vi "Dresden R2R Sputter 03.02.2018 IY24.vi"() -> ()   [LabVIEW 2009] (continued)
                                n16803 = local write "Semi"(TRUE ("Semi")) -> ()
                                }
                                }
                                n16804 = local read "Ch1_Ch_atm_di"() -> (w27011:bool)
                                n16805 = case shown="False" w27011 {
                                tunnel: [w27018 TRUE] -> w27013
                                frame #0 {
                                n16806 = local read "Ch1_Ch_vbv_di"() -> (w27019:bool)
                                n16807 = case shown="False" w27019 {
                                tunnel: [FALSE TRUE] -> w27018
                                frame #0 {
                                n16808 = Wait Until Next ms Multiple(millisecond multiple=u32 200) -> ()  [unwired: 1 out]
                                n16809 = local write "Ch1_Ch_vbv_do"(TRUE ("Ch1_Ch_cc_on_off_di")) -> ()
                                }
                                frame #1 {
                                }
                                }
                                }
                                frame #1 {
                                }
                                }
                                n16810 = local read "Semi"() -> (w27014:bool)
                                n16811 = Or(x=w27013, y=w27014) -> (x .or. y?=w27012:bool)
                                }
                                }
                                frame #1 {
                                }
                                }
                                }
                                frame #2 {
                                n16812 = local read "Semi"() -> (w27027:bool)
                                n16813 = case shown="False" w27027 {
                                frame #0 {
                                n16814 = local write "Ch1_Sd10"(TRUE ("Ch1_Sd9")) -> ()
                                n16815 = Wait (ms)(milliseconds to wait=u32 1000) -> ()  [unwired: 1 out]
                                }
                                frame #1 {
                                }
                                }
                                }
                                }
                                }
                                frame #1 {
                                }
                                }
                                }
                                }
                              }
                              frame #11 {
                                # "CH-VBV CLOSE &  CHECK"
                                n16816 = local read "Yes"() -> (w27030:bool)
                                n16817 = case shown="True" w27030 {
                                frame #0 {
                                }
                                frame #1 {
                                n16818 = local read "Semi"() -> (w27031:bool)
                                n16819 = case shown="False" w27031 {
                                frame #0 {
                                n16820 = stacked-sequence {
                                frame #0 {
                                n16821 = local read "Semi"() -> (w27032:bool)
                                n16822 = case shown="False" w27032 {
                                frame #0 {
                                n16823 = while {
                                i -> [w27040]
                                stop <- w27036 stop-if-true
                                n16824 = Greater?(x=w27040, y=50) -> (0:w27039:bool)
                                n16825 = case shown="True" w27039 {
                                frame #0 {
                                }
                                frame #1 {
                                n16826 = local write "Error Message"("Shut Down Process  cancelled\nbecause  CH-VBV  not closed.\nPlease check CH-VBV1 connections." ("Error Message")) -> ()
                                n16827 = local write "Semi"(TRUE ("Semi")) -> ()
                                }
                                }
                                n16828 = local read "Tp1_speed_gui"() -> (w27034:i32)
                                n16829 = Greater Or Equal?(x=w27034, y=u64 100) -> (x >= y?=w27033:bool)
                                n16830 = case shown="True" w27033 {
                                tunnel: [TRUE w27043] -> w27037
                                frame #0 {
                                }
                                frame #1 {
                                n16831 = local read "Ch1_Ch_vbv_di"() -> (w27044:bool)
                                n16832 = case shown="True" w27044 {
                                tunnel: [TRUE FALSE] -> w27043
                                frame #0 {
                                }
                                frame #1 {
                                n16833 = Wait Until Next ms Multiple(millisecond multiple=u32 500) -> ()  [unwired: 1 out]
                                n16834 = local write "Ch1_Ch_vbv_do"(FALSE ("Ch1_Ch_cc_on_off_di")) -> ()
                                }
                                }
                                }
                                }
                                n16835 = local read "Semi"() -> (w27038:bool)
                                n16836 = Or(x=w27037, y=w27038) -> (x .or. y?=w27036:bool)
                                }
                                }
                                frame #1 {
                                }
                                }
                                }
                                frame #1 {
                                n16837 = local read "Semi"() -> (w27051:bool)
                                n16838 = case shown="False" w27051 {
                                frame #0 {
                                n16839 = local write "Ch1_Sd11"(TRUE ("Ch1_Sd13")) -> ()
                                n16840 = Wait (ms)(milliseconds to wait=u32 1000) -> ()  [unwired: 1 out]
                                }
                                frame #1 {
                                }
                                }
                                }
                                frame #2 {
                                n16841 = local read "Semi"() -> (w27054:bool)
                                n16842 = case shown="False" w27054 {
                                frame #0 {
                                n16843 = Wait (ms)(milliseconds to wait=u32 3000) -> ()  [unwired: 1 out]
                                }
                                frame #1 {
                                }
                                }
                                }
                                }
                                }
                                frame #1 {
                                }
                                }
                                }
                                }
                              }
                              frame #12 {
                                # "CH-VBV OPEN &  CHECK"
                                n16844 = local read "Yes"() -> (w27056:bool)
                                n16845 = case shown="True" w27056 {
                                frame #0 {
                                }
                                frame #1 {
                                n16846 = local read "Semi"() -> (w27057:bool)
                                n16847 = case shown="False" w27057 {
                                frame #0 {
                                n16848 = stacked-sequence {
                                frame #0 {
                                n16849 = local read "Semi"() -> (w27058:bool)
                                n16850 = case shown="False" w27058 {
                                frame #0 {
                                n16851 = while {
                                i -> [w27064]
                                stop <- w27060 stop-if-true
                                n16852 = Greater?(x=w27064, y=200) -> (0:w27063:bool)
                                n16853 = case shown="True" w27063 {
                                frame #0 {
                                }
                                frame #1 {
                                n16854 = local write "Error Message"("Shut Down Process  cancelled\nbecause  CH-VBV  not opened.\nPlease check CH-VBV1 connections." ("Error Message")) -> ()
                                n16855 = local write "Semi"(TRUE ("Semi")) -> ()
                                }
                                }
                                n16856 = local read "Ch1_Ch_vbv_di"() -> (w27059:bool)
                                n16857 = case shown="False" w27059 {
                                tunnel: [FALSE TRUE] -> w27061
                                frame #0 {
                                n16858 = local write "Ch1_Ch_vbv_do"(TRUE ("Ch1_Ch_cc_on_off_di")) -> ()
                                n16859 = Wait Until Next ms Multiple(millisecond multiple=u32 500) -> ()  [unwired: 1 out]
                                }
                                frame #1 {
                                }
                                }
                                n16860 = local read "Semi"() -> (w27062:bool)
                                n16861 = Or(x=w27061, y=w27062) -> (x .or. y?=w27060:bool)
                                }
                                }
                                frame #1 {
                                }
                                }
                                }
                                frame #1 {
                                n16862 = local read "Semi"() -> (w27072:bool)
                                n16863 = case shown="False" w27072 {
                                frame #0 {
                                n16864 = local write "Ch1_Sd12"(TRUE ("Ch1_Sd12")) -> ()
                                n16865 = Wait (ms)(milliseconds to wait=u32 1000) -> ()  [unwired: 1 out]
                                }
                                frame #1 {
                                }
                                }
                                }
                                }
                                }
                                frame #1 {
                                }
                                }
                                }
                                }
                              }
                              frame #13 {
                                # "TRNS GV-BP2 OPEN"
                                n16866 = local read "Yes"() -> (w27075:bool)
                                n16867 = case shown="True" w27075 {
                                frame #0 {
                                }
                                frame #1 {
                                n16868 = local read "Semi"() -> (w27076:bool)
                                n16869 = case shown="False" w27076 {
                                frame #0 {
                                n16870 = stacked-sequence {
                                frame #0 {
                                n16871 = local read "Semi"() -> (w27077:bool)
                                n16872 = case shown="False" w27077 {
                                frame #0 {
                                n16873 = while {
                                i -> [w27085]
                                stop <- w27082 stop-if-true
                                n16874 = Greater?(x=w27085, y=800) -> (0:w27084:bool)
                                n16875 = case shown="True" w27084 {
                                frame #0 {
                                }
                                frame #1 {
                                n16876 = local write "Error Message"("Shut Down process was cancelled.\nPlease check Trns GV-BP2\n connections." ("Error Message")) -> ()
                                n16877 = local write "Semi"(TRUE ("Semi")) -> ()
                                }
                                }
                                n16878 = local read "Ch1_pressure"() -> (w27080:dbl)
                                n16879 = Greater Or Equal?(x=w27080, y=700.0) -> (x >= y?=w27078:bool)
                                n16880 = case shown="False" w27078 {
                                tunnel: [FALSE w27089] -> w27081
                                frame #0 {
                                n16881 = Wait Until Next ms Multiple(millisecond multiple=u32 500) -> ()  [unwired: 1 out]
                                }
                                frame #1 {
                                n16882 = local read "Ch1_Trns_gv_bp2_di"() -> (w27090:bool)
                                n16883 = case shown="False" w27090 {
                                tunnel: [FALSE TRUE] -> w27089
                                frame #0 {
                                n16884 = local write "Ch1_Trns_gv_bp2_do"(TRUE ("Ch1_Trns_gv_bp2_do")) -> ()
                                n16885 = Wait Until Next ms Multiple(millisecond multiple=u32 500) -> ()  [unwired: 1 out]
                                }
                                frame #1 {
                                }
                                }
                                }
                                }
                                n16886 = local read "Semi"() -> (w27083:bool)
                                n16887 = Or(x=w27081, y=w27083) -> (x .or. y?=w27082:bool)
                                }
                                }
                                frame #1 {
                                }
                                }
                                }
                                frame #1 {
                                n16888 = local read "Semi"() -> (w27097:bool)
                                n16889 = case shown="False" w27097 {
                                frame #0 {
                                n16890 = Wait (ms)(milliseconds to wait=u32 1000) -> ()  [unwired: 1 out]
                                n16891 = local write "Ch1_Sd13"(TRUE ("Ch1_Sd12")) -> ()
                                }
                                frame #1 {
                                }
                                }
                                }
                                frame #2 {
                                n16892 = local read "Semi"() -> (w27100:bool)
                                n16893 = case shown="False" w27100 {
                                frame #0 {
                                n16894 = Wait (ms)(milliseconds to wait=u32 2000) -> ()  [unwired: 1 out]
                                }
                                frame #1 {
                                }
                                }
                                }
                                }
                                }
                                frame #1 {
                                }
                                }
                                }
                                }
                              }
                              frame #14 {
                                # "CH-ATM OPEN &  CHECK"
                                n16895 = local read "Yes"() -> (w27102:bool)
                                n16896 = case shown="True" w27102 {
                                frame #0 {
                                }
                                frame #1 {
                                n16897 = local read "Semi"() -> (w27103:bool)
                                n16898 = case shown="False" w27103 {
                                frame #0 {
                                n16899 = stacked-sequence {
                                frame #0 {
                                n16900 = local read "Semi"() -> (w27104:bool)
                                n16901 = case shown="False" w27104 {
                                frame #0 {
                                n16902 = while {
                                i -> [w27110]
                                stop <- w27107 stop-if-true
                                n16903 = Greater?(x=w27110, y=1700) -> (0:w27109:bool)
                                n16904 = case shown="True" w27109 {
                                frame #0 {
                                }
                                frame #1 {
                                n16905 = local write "Error Message"("Shut Down process was cancelled.\nPlease check Chamber \nvacuum connections." ("Error Message")) -> ()
                                n16906 = local write "Semi"(TRUE ("Semi")) -> ()
                                }
                                }
                                n16907 = local read "Ch1_Ch_atm_di"() -> (w27106:bool)
                                n16908 = case shown="False" w27106 {
                                tunnel: [FALSE TRUE] -> w27105
                                frame #0 {
                                n16909 = Wait Until Next ms Multiple(millisecond multiple=u32 500) -> ()  [unwired: 1 out]
                                }
                                frame #1 {
                                }
                                }
                                n16910 = local read "Semi"() -> (w27108:bool)
                                n16911 = Or(x=w27105, y=w27108) -> (x .or. y?=w27107:bool)
                                }
                                }
                                frame #1 {
                                }
                                }
                                }
                                frame #1 {
                                n16912 = local read "Semi"() -> (w27117:bool)
                                n16913 = case shown="False" w27117 {
                                frame #0 {
                                n16914 = local write "Ch1_Sd14"(TRUE ("Ch1_Sd10")) -> ()
                                n16915 = Wait (ms)(milliseconds to wait=u32 1000) -> ()  [unwired: 1 out]
                                }
                                frame #1 {
                                }
                                }
                                }
                                frame #2 {
                                n16916 = local read "Semi"() -> (w27120:bool)
                                n16917 = case shown="False" w27120 {
                                frame #0 {
                                n16918 = Wait (ms)(milliseconds to wait=u32 2000) -> ()  [unwired: 1 out]
                                }
                                frame #1 {
                                }
                                }
                                }
                                }
                                }
                                frame #1 {
                                }
                                }
                                }
                                }
                              }
                              frame #15 {
                                # "TRNS GV-BP2 OPEN"
                                n16919 = local read "Semi"() -> (w27122:bool)
                                n16920 = case shown="False" w27122 {
                                frame #0 {
                                n16921 = stacked-sequence {
                                frame #0 {
                                n16922 = local read "Semi"() -> (w27123:bool)
                                n16923 = case shown="False" w27123 {
                                frame #0 {
                                n16924 = while {
                                i -> [w27129]
                                stop <- w27125 stop-if-true
                                n16925 = Greater?(x=w27129, y=50) -> (0:w27128:bool)
                                n16926 = case shown="True" w27128 {
                                frame #0 {
                                }
                                frame #1 {
                                n16927 = local write "Error Message"("Shut Down Process  cancelled\nbecause  Trns-GV-BP2  not closed.\nPlease check Trns-GV-BP2  connections." ("Error Message")) -> ()
                                n16928 = local write "Semi"(TRUE ("Semi")) -> ()
                                }
                                }
                                n16929 = local read "Ch1_Trns_gv_bp2_di"() -> (w27124:bool)
                                n16930 = case shown="True" w27124 {
                                tunnel: [TRUE FALSE] -> w27126
                                frame #0 {
                                }
                                frame #1 {
                                n16931 = Wait Until Next ms Multiple(millisecond multiple=u32 500) -> ()  [unwired: 1 out]
                                n16932 = local write "Ch1_Trns_gv_bp2_do"(FALSE ("Ch1_Ch_cc_on_off_di")) -> ()
                                }
                                }
                                n16933 = local read "Semi"() -> (w27127:bool)
                                n16934 = Or(x=w27126, y=w27127) -> (x .or. y?=w27125:bool)
                                }
                                }
                                frame #1 {
                                }
                                }
                                }
                                frame #1 {
                                n16935 = local read "Semi"() -> (w27137:bool)
                                n16936 = case shown="False" w27137 {
                                frame #0 {
                                n16937 = local write "Ch1_Sd15"(TRUE ("Ch1_Sd10 3")) -> ()
                                n16938 = Wait (ms)(milliseconds to wait=u32 1000) -> ()  [unwired: 1 out]
                                }
                                frame #1 {
                                }
                                }
                                }
                                }
                                }
                                frame #1 {
                                }
                                }
                              }
                              frame #16 {
                                # "CH-VBV CLOSE &  CHECK"
                                n16939 = local read "Yes"() -> (w27140:bool)
                                n16940 = case shown="True" w27140 {
                                frame #0 {
                                }
                                frame #1 {
                                n16941 = local read "Semi"() -> (w27141:bool)
                                n16942 = case shown="False" w27141 {
                                frame #0 {
                                n16943 = stacked-sequence {
                                frame #0 {
                                n16944 = local read "Semi"() -> (w27142:bool)
                                n16945 = case shown="False" w27142 {
                                frame #0 {
                                n16946 = while {
                                i -> [w27152]
                                stop <- w27148 stop-if-true
                                n16947 = Greater?(x=w27152, y=50) -> (0:w27151:bool)
                                n16948 = case shown="True" w27151 {
                                frame #0 {
                                }
                                frame #1 {
                                n16949 = local write "Error Message"("Shut Down Process  cancelled\nbecause  CH-VBV  not closed.\nPlease check CH-VBV1 connections." ("Error Message")) -> ()
                                n16950 = local write "Semi"(TRUE ("Semi")) -> ()
                                }
                                }
                                n16951 = local read "Tp1_speed_gui"() -> (w27146:i32)
                                n16952 = local read "Yes"() -> (w27145:bool)
                                n16953 = Greater Or Equal?(x=w27146, y=u64 100) -> (x >= y?=w27144:bool)
                                n16954 = And(x=w27145, y=w27144) -> (x .and. y?=w27143:bool)
                                n16955 = case shown="True" w27143 {
                                tunnel: [TRUE w27155] -> w27149
                                frame #0 {
                                }
                                frame #1 {
                                n16956 = local read "Ch1_Ch_vbv_di"() -> (w27156:bool)
                                n16957 = case shown="False" w27156 {
                                tunnel: [TRUE FALSE] -> w27155
                                frame #0 {
                                }
                                frame #1 {
                                n16958 = Wait Until Next ms Multiple(millisecond multiple=u32 500) -> ()  [unwired: 1 out]
                                n16959 = local write "Ch1_Ch_vbv_do"(FALSE ("Ch1_Ch_cc_on_off_di")) -> ()
                                }
                                }
                                }
                                }
                                n16960 = local read "Semi"() -> (w27150:bool)
                                n16961 = Or(x=w27149, y=w27150) -> (x .or. y?=w27148:bool)
                                }
                                }
                                frame #1 {
                                }
                                }
                                }
                                frame #1 {
                                n16962 = local read "Semi"() -> (w27163:bool)
                                n16963 = case shown="False" w27163 {
                                frame #0 {
                                n16964 = local write "Ch1_Sd16"(TRUE ("Ch1_Sd10 2")) -> ()
                                n16965 = Wait (ms)(milliseconds to wait=u32 1000) -> ()  [unwired: 1 out]
                                }
                                frame #1 {
                                }
                                }
                                }
                                frame #2 {
                                n16966 = local read "Semi"() -> (w27166:bool)
                                n16967 = case shown="False" w27166 {
                                frame #0 {
                                n16968 = Wait (ms)(milliseconds to wait=u32 3000) -> ()  [unwired: 1 out]
                                }
                                frame #1 {
                                }
                                }
                                }
                                }
                                }
                                frame #1 {
                                }
                                }
                                }
                                }
                              }
                              frame #17 {
                                # "CLOSE PC-BV"
                                n16969 = local read "Yes"() -> (w27168:bool)
                                n16970 = case shown="True" w27168 {
                                frame #0 {
                                }
                                frame #1 {
                                n16971 = local read "Semi"() -> (w27169:bool)
                                n16972 = case shown="False" w27169 {
                                frame #0 {
                                n16973 = stacked-sequence {
                                frame #0 {
                                n16974 = local read "Semi"() -> (w27170:bool)
                                n16975 = case shown="False" w27170 {
                                frame #0 {
                                n16976 = stacked-sequence {
                                frame #0 {
                                n16977 = local read "Semi"() -> (w27171:bool)
                                n16978 = case shown="False" w27171 {
                                frame #0 {
                                n16979 = local write "Pc_bv1_auto_close"(TRUE ("Tp1_auto_start")) -> ()
                                }
                                frame #1 {
                                }
                                }
                                }
                                frame #1 {
                                n16980 = local read "Semi"() -> (w27173:bool)
                                n16981 = case shown="False" w27173 {
                                frame #0 {
                                n16982 = Wait (ms)(milliseconds to wait=u32 1000) -> ()  [unwired: 1 out]
                                }
                                frame #1 {
                                }
                                }
                                }
                                frame #2 {
                                n16983 = local read "Semi"() -> (w27175:bool)
                                n16984 = case shown="False" w27175 {
                                frame #0 {
                                n16985 = while {
                                i -> [w27181]
                                stop <- w27177 stop-if-true
                                n16986 = local read "Pc_bv_closed_ch1"() -> (w27179:bool)
                                n16987 = Greater?(x=w27181, y=120) -> (0:w27180:bool)
                                n16988 = local read "Semi"() -> (w27178:bool)
                                n16989 = Compound Arithmetic op=OR(w27178, w27179, w27180) -> (w27177:bool)
                                n16990 = Wait (ms)(milliseconds to wait=u32 500) -> ()  [unwired: 1 out]
                                }
                                }
                                frame #1 {
                                }
                                }
                                }
                                frame #3 {
                                n16991 = local read "Semi"() -> (w27183:bool)
                                n16992 = case shown="False" w27183 {
                                frame #0 {
                                n16993 = local read "Pc_bv_closed_ch1"() -> (w27184:bool)
                                n16994 = case shown="False" w27184 {
                                frame #0 {
                                n16995 = local write "Pc_bv1_auto_close"(TRUE ("Pc_bv1_auto_open")) -> ()
                                }
                                frame #1 {
                                }
                                }
                                }
                                frame #1 {
                                }
                                }
                                }
                                frame #4 {
                                n16996 = local read "Semi"() -> (w27186:bool)
                                n16997 = case shown="False" w27186 {
                                frame #0 {
                                n16998 = local read "Pc_bv_closed_ch1"() -> (w27187:bool)
                                n16999 = case shown="False" w27187 {
                                frame #0 {
                                n17000 = Wait (ms)(milliseconds to wait=u32 1000) -> ()  [unwired: 1 out]
                                }
                                frame #1 {
                                }
                                }
                                }
                                frame #1 {
                                }
                                }
                                }
                                frame #5 {
                                n17001 = local read "Semi"() -> (w27189:bool)
                                n17002 = case shown="False" w27189 {
                                frame #0 {
                                n17003 = while {
                                i -> [w27195]
                                stop <- w27191 stop-if-true
                                n17004 = local read "Pc_bv_closed_ch1"() -> (w27193:bool)
                                n17005 = Greater?(x=w27195, y=120) -> (0:w27194:bool)
                                n17006 = local read "Semi"() -> (w27192:bool)
                                n17007 = Compound Arithmetic op=OR(w27192, w27193, w27194) -> (w27191:bool)
                                n17008 = Wait (ms)(milliseconds to wait=u32 500) -> ()  [unwired: 1 out]
                                }
                                }
                                frame #1 {
                                }
                                }
                                }
                                frame #6 {
                                n17009 = local read "Semi"() -> (w27197:bool)
                                n17010 = case shown="False" w27197 {
                                frame #0 {
                                n17011 = local read "Pc_bv_closed_ch1"() -> (w27198:bool)
                                n17012 = case shown="False" w27198 {
                                frame #0 {
                                n17013 = local write "Error Message"("Shut Down process  cancelled\nbecause  PC-BV not closed.\nPlease check PC-BV1 connections." ("Error Message")) -> ()
                                n17014 = Wait (ms)(milliseconds to wait=u32 1000) -> ()  [unwired: 1 out]
                                }
                                frame #1 {
                                }
                                }
                                }
                                frame #1 {
                                }
                                }
                                }
                                }
                                }
                                frame #1 {
                                }
                                }
                                }
                                frame #1 {
                                n17015 = local read "Semi"() -> (w27201:bool)
                                n17016 = case shown="False" w27201 {
                                frame #0 {
                                n17017 = Wait (ms)(milliseconds to wait=u32 1000) -> ()  [unwired: 1 out]
                                n17018 = local write "Ch1_Sd17"(TRUE ("Ch1_Sd14")) -> ()
                                }
                                frame #1 {
                                }
                                }
                                }
                                }
                                }
                                frame #1 {
                                }
                                }
                                }
                                }
                              }
                              frame #18 {
                                # "CH-VBV CLOSE &  CHECK"
                                n17019 = local read "Semi"() -> (w27204:bool)
                                n17020 = case shown="False" w27204 {
                                frame #0 {
                                n17021 = stacked-sequence {
                                frame #0 {
                                n17022 = local read "Semi"() -> (w27205:bool)
                                n17023 = case shown="False" w27205 {
                                frame #0 {
                                n17024 = while {
                                i -> [w27211]
                                stop <- w27207 stop-if-true
                                n17025 = Greater?(x=w27211, y=50) -> (0:w27210:bool)
                                n17026 = case shown="True" w27210 {
                                frame #0 {
                                }
                                frame #1 {
                                n17027 = local write "Error Message"("Shut Down Process  cancelled\nbecause  CH-VBV  not closed.\nPlease check CH-VBV1 connections." ("Error Message")) -> ()
                                n17028 = local write "Semi"(TRUE ("Semi")) -> ()
                                }
                                }
                                n17029 = local read "Ch1_Ch_vbv_di"() -> (w27206:bool)
                                n17030 = case shown="True" w27206 {
                                tunnel: [TRUE FALSE] -> w27208
                                frame #0 {
                                }
                                frame #1 {
                                n17031 = Wait Until Next ms Multiple(millisecond multiple=u32 500) -> ()  [unwired: 1 out]
                                n17032 = local write "Ch1_Ch_vbv_do"(FALSE ("Ch1_Ch_cc_on_off_di")) -> ()
                                }
                                }
                                n17033 = local read "Semi"() -> (w27209:bool)
                                n17034 = Or(x=w27208, y=w27209) -> (x .or. y?=w27207:bool)
                                }
                                }
                                frame #1 {
                                }
                                }
                                }
                                frame #1 {
                                n17035 = local read "Semi"() -> (w27219:bool)
                                n17036 = case shown="False" w27219 {
                                frame #0 {
                                n17037 = local write "Ch1_Sd18"(TRUE ("Ch1_Sd10 3")) -> ()
                                n17038 = Wait (ms)(milliseconds to wait=u32 1000) -> ()  [unwired: 1 out]
                                }
                                frame #1 {
                                }
                                }
                                }
                                }
                                }
                                frame #1 {
                                }
                                }
                              }
                              frame #19 {
                                # "FINISH SHUTDOWN"
                                n17039 = local read "Semi"() -> (w27222:bool)
                                n17040 = case shown="False" w27222 {
                                frame #0 {
                                n17041 = stacked-sequence {
                                frame #0 {
                                n17042 = local read "Semi"() -> (w27223:bool)
                                n17043 = case shown="False" w27223 {
                                frame #0 {
                                w27224 = TRUE ("Visible")
                                n17044 = property on="final_mes_tab" class="TabCtl (strict)"("Visible"=w27224) -> ()  [unwired: 2 in, 2 out]
                                n17045 = local write "Cnt_Do_Buzzer"(w27224) -> ()
                                n17046 = local write "system_status"("Shut Down Process was completed." ("system_status")) -> ()
                                n17047 = Wait (ms)(milliseconds to wait=u32 3000) -> ()  [unwired: 1 out]
                                }
                                frame #1 {
                                }
                                }
                                }
                                frame #1 {
                                n17048 = local read "Semi"() -> (w27227:bool)
                                n17049 = case shown="False" w27227 {
                                frame #0 {
                                w27230 = FALSE ("Visible")
                                n17050 = property on="final_mes_tab" class="TabCtl (strict)"("Visible"=w27230) -> ()  [unwired: 2 in, 2 out]
                                n17051 = local write "Shutdown_ch1"(w27230) -> ()
                                n17052 = local write "Cnt_Do_Buzzer"(w27230) -> ()
                                n17053 = local write "system_status"("" ("system_status")) -> ()
                                n17054 = Wait (ms)(milliseconds to wait=u32 3000) -> ()  [unwired: 1 out]
                                }
                                frame #1 {
                                }
                                }
                                }
                                frame #2 {
                                n17055 = local read "Semi"() -> (w27231:bool)
                                n17056 = case shown="False" w27231 {
                                frame #0 {
                                n17057 = stacked-sequence {
                                frame #0 {
                                n17058 = local write "Pps_code_entry"("PF233=" ("Pps_code_entry")) -> ()
                                }
                                frame #1 {
                                n17059 = Wait (ms)(milliseconds to wait=u32 500) -> ()  [unwired: 1 out]
                                }
                                frame #2 {
                                n17060 = local write "Ppsok"(TRUE ("Ppsok")) -> ()
                                }
                                frame #3 {
                                n17061 = Wait (ms)(milliseconds to wait=u32 500) -> ()  [unwired: 1 out]
                                }
                                }
                                }
                                frame #1 {
                                }
                                }
                                }
                                frame #3 {
                                n17062 = local read "Semi"() -> (w27236:bool)
                                n17063 = case shown="False" w27236 {
                                frame #0 {
                                n17064 = stacked-sequence {
                                frame #0 {
                                n17065 = local write "Pps_code_entry"("PF234=" ("Pps_code_entry")) -> ()
                                }
                                frame #1 {
                                n17066 = Wait (ms)(milliseconds to wait=u32 500) -> ()  [unwired: 1 out]
                                }
                                frame #2 {
                                n17067 = local write "Ppsok"(TRUE ("Ppsok")) -> ()
                                }
                                frame #3 {
                                n17068 = Wait (ms)(milliseconds to wait=u32 500) -> ()  [unwired: 1 out]
                                }
                                }
                                }
                                frame #1 {
                                }
                                }
                                }
                                frame #4 {
                                n17069 = local read "Semi"() -> (w27241:bool)
                                n17070 = case shown="False" w27241 {
                                frame #0 {
                                n17071 = local write "Ch1_Sd19"(TRUE ("Ch1_Sd15")) -> ()
                                n17072 = Wait (ms)(milliseconds to wait=u32 500) -> ()  [unwired: 1 out]
                                }
                                frame #1 {
                                }
                                }
                                }
                                }
                                }
                                frame #1 {
                                }
                                }
                              }
                            }
                          }
                        }
                      }
                    }
                  }
                  frame #1 {
                  }
                }
              }
            }
          }
          frame #1 {
          }
        }
      }
    }
    n17073 = Wait Until Next ms Multiple(millisecond multiple=i32? 300) -> ()  [unwired: 1 out]
    n17074 = case shown="True" "Start_up_ch2" {
      frame #0 {
      }
      frame #1 {
        # "START UP OF CH2 PROCEDURE"
        n17075 = stacked-sequence {
          frame #0 {
            # "ROUTINE CHECK"
            n17076 = local read "Semi"() -> (w25558:bool)
            n17077 = case shown="False" w25558 {
              frame #0 {
                n17078 = stacked-sequence {
                  frame #0 {
                    n17079 = local write "Clean_Pumping_ch2"(TRUE) -> ()
                    n17080 = property on="Pressure_time_graph_ch2" class="WFChart (strict)"("History Data"=dbl[] []) -> ()  [unwired: 2 in, 2 out]
                    n17081 = local write "final_process_messages"("Start up process was completed." ("final_process_messages")) -> ()
                    n17082 = local write "system_status"("Start up process continues." ("system_status")) -> ()
                    n17083 = Wait (ms)(milliseconds to wait=u32 1000) -> ()  [unwired: 1 out]
                  }
                  frame #1 {